vi "test33.vi"() -> ()   [LabVIEW 2021]
uses:
  fft -- waveform manipulate -- control.vi.ctl
  aggregator - viii - real - atomic.vi
  linear interp iiii- real - z-omega.vi
  linear interpolation - real -- V2.vi
  <vilib>/Analysis/baseanly.llb/A x B.vi
  <vilib>/Analysis/baseanly.llb/Real A x B.vi
  Q -- check range -- i -- real.vi
  line -- complex.vi
  Q -- check range -- i -- integer.vi
  Q - not nan -- real.vi
  Q - not nan -- integer.vi
  <vilib>/gmath/interp.llb/Interpolate 1D.vi
  <vilib>/gmath/interp.llb/Search Ordered Table.vi
  <vilib>/Analysis/Matrix/Numeric/Conversions/Array To Matrix.vi
  <vilib>/Analysis/Matrix/Numeric/Conversions/Array To Matrix - RA2.vi
  <vilib>/Analysis/baseanly.llb/Inverse Matrix.vi
  <vilib>/Analysis/baseanly.llb/Real Inverse Matrix.vi
panel:
  in  "times":dbl[](array[numeric]) format="%#_3p"
  out "size(s) 5":i32
  out "size(s) 6":i32
  out "freq vs time 5":cluster{dbl[], dbl[]}(graph)
  out "Array 6":dbl[](array[numeric]) format="%#_3p"
  out "Array 5":dbl[](array[numeric]) format="%#_3p"
  out "freq vs time 4":cluster{dbl[], dbl[]}(graph)
  out "size(s) 3":i32
  out "size(s) 4":i32
  out "Array 4":dbl[](array[numeric]) format="%#_3p"
  out "Array 3":dbl[](array[numeric]) format="%#_3p"
  out "size(s)":i32
  out "size(s) 2":i32
  out "freq vs time 3":cluster{dbl[], dbl[]}[](graph)
  out "Array 2":dbl[](array[numeric]) format="%#_3p"
  out "Array":dbl[](array[numeric]) format="%#_3p"
  out "freq vs time 2":cluster{dbl[], dbl[]}(graph)
  in  "field vs time":cluster{dbl[], dbl[]}(graph)={array[333333 elements], array[333333 elements]}
  in  "freq vs time":cluster{dbl[], dbl[]}(graph)={array[2402 elements], array[2402 elements]}
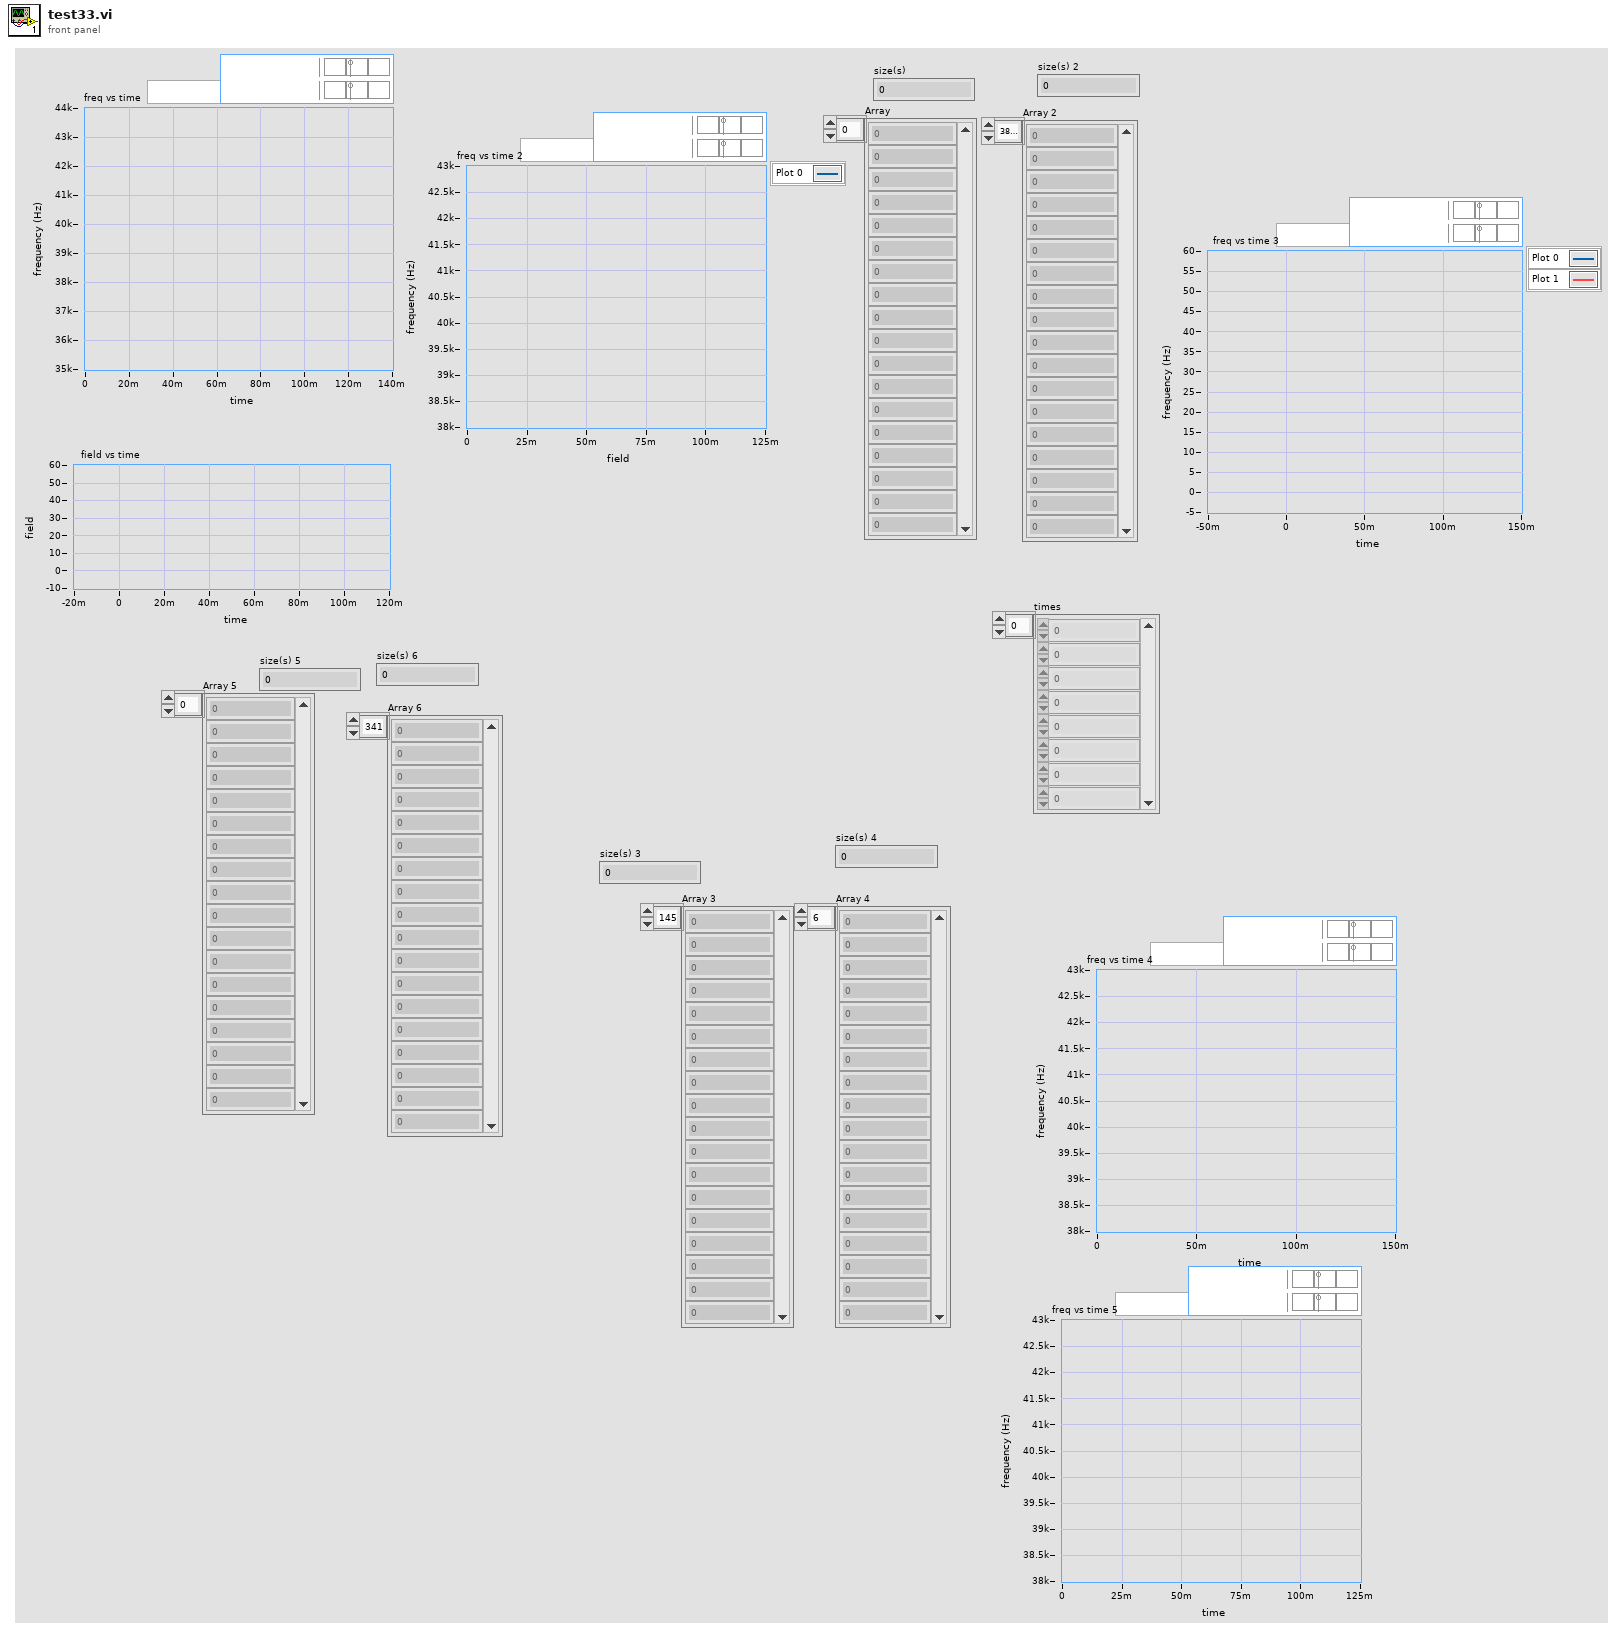
[diagram p1: front panel]
types:
  T1 = typedef "fft -- waveform manipulate -- control.vi.ctl" = enum16{"to array", "to map", "ref from map", "interp from map", "interp from array", "interp other", "delay", "get gamma", "clean 1", "clean 2"}
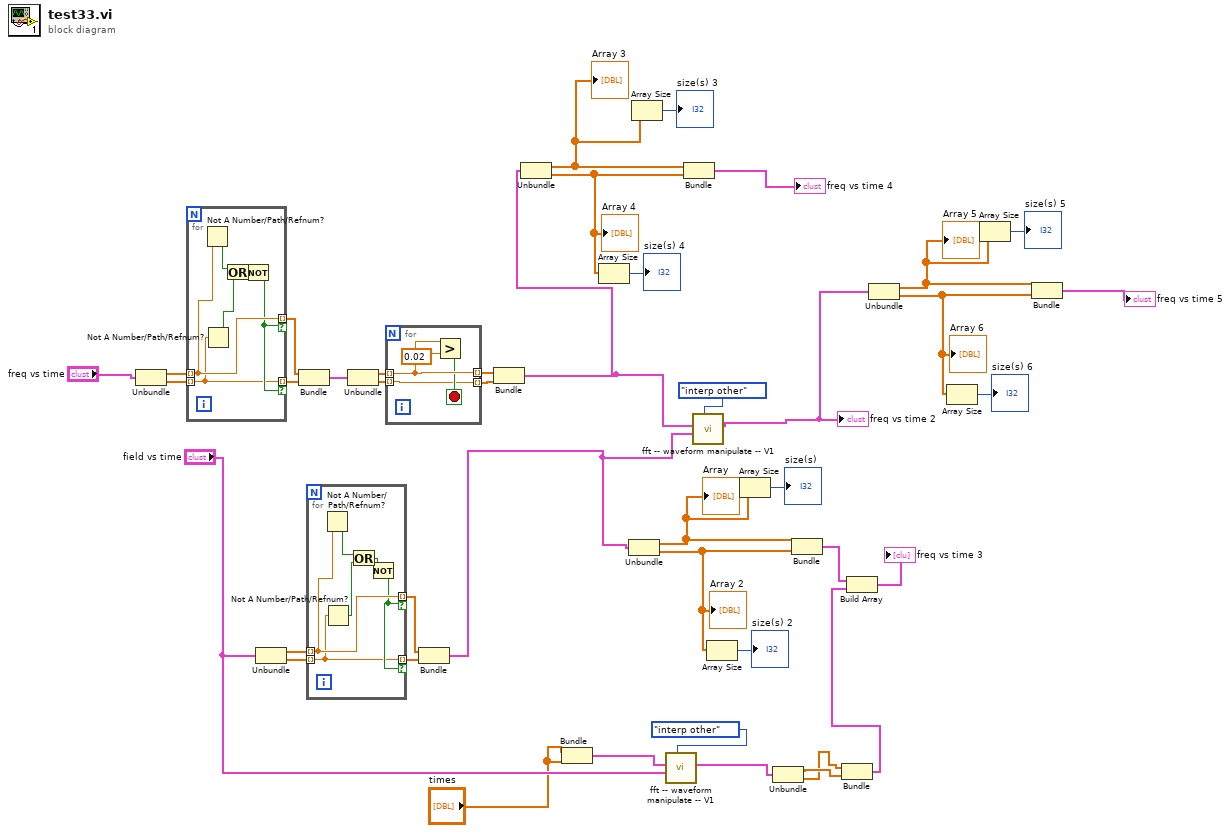
[diagram p0: block diagram]
diagram:
  n1 = Unbundle("freq vs time") -> (w31:dbl[], w30:dbl[])
  n2 = for {
    tunnel: w31 -> [w48] mode=indexing
    tunnel: w30 -> [w43] mode=indexing
    tunnel: [w48] -> w29 mode=indexing if=w44
    tunnel: [w43] -> w28 mode=indexing if=w44
    n3 = Not A Number/Path/Refnum?(number/path/refnum=w48) -> (NaN/Path/Refnum?=w47:bool)
    n4 = Not A Number/Path/Refnum?(number/path/refnum=w43) -> (NaN/Path/Refnum?=w46:bool)
    n5 = Or(x=w47, y=w46) -> (x .or. y?=w45:bool)
    n6 = Not(x=w45) -> (.not. x?=w44:bool)
  }
  n7 = Unbundle("field vs time") -> (w27:dbl[], w26:dbl[])
  n8 = Bundle(w29, w28) -> (w16:cluster{dbl[], dbl[]})  [unwired: 1 in]
  n9 = for {
    tunnel: w27 -> [w54] mode=indexing
    tunnel: w26 -> [w49] mode=indexing
    tunnel: [w54] -> w25 mode=indexing if=w50
    tunnel: [w49] -> w24 mode=indexing if=w50
    n10 = Not A Number/Path/Refnum?(number/path/refnum=w54) -> (NaN/Path/Refnum?=w53:bool)
    n11 = Not A Number/Path/Refnum?(number/path/refnum=w49) -> (NaN/Path/Refnum?=w52:bool)
    n12 = Or(x=w53, y=w52) -> (x .or. y?=w51:bool)
    n13 = Not(x=w51) -> (.not. x?=w50:bool)
  }
  n14 = Unbundle(w16) -> (w15:dbl[], w12:dbl[])
  n15 = for {
    tunnel: [w58] -> w14 mode=indexing
    tunnel: w15 -> [w58] mode=indexing
    tunnel: [w55] -> w13 mode=indexing
    tunnel: w12 -> [w55] mode=indexing
    stop <- w56 stop-if-true
    n16 = Greater?(x=w58, y=0.02) -> (0:w56:bool)
  }
  n17 = Bundle(w25, w24) -> (w23:cluster{dbl[], dbl[]})  [unwired: 1 in]
  n18 = Bundle(w14, w13) -> (w11:cluster{dbl[], dbl[]})  [unwired: 1 in]
  n19 = Unbundle(w11) -> (w34:dbl[], w37:dbl[])
  "Array 3" <- w34
  "Array 4" <- w37
  n20 = Bundle("times"="times", "times"="times") -> (w9:cluster{"times":dbl[], "times":dbl[]})  [unwired: 1 in]
  n21 = Array Size(array=w37) -> (size(s)=→"size(s) 4":i32)
  n22 = Unbundle(w23) -> (w38:dbl[], w41:dbl[])
  "Array" <- w38
  "Array 2" <- w41
  n23 = Array Size(array=w34) -> (size(s)=→"size(s) 3":i32)
  n24 = call "fft -- waveform manipulate -- V1.vi"("fft -- manipulate"=fft_--_waveform_manipulate_--_control.vi."interp other", "Ref Cluster IN"="field vs time", "Cluster IN"=w9) -> ("Cluster out"=w5:cluster{dbl[], dbl[]})  [unwired: 5 in, 3 out]
  n25 = Bundle(w34, w37) -> (→"freq vs time 4":cluster{dbl[], dbl[]})  [unwired: 1 in]
  n26 = call "fft -- waveform manipulate -- V1.vi"("fft -- manipulate"=fft_--_waveform_manipulate_--_control.vi."interp other", "Ref Cluster IN"=w23, "Cluster IN"=w11) -> ("Cluster out"=w17:cluster{dbl[], dbl[]})  [unwired: 5 in, 3 out]
  "freq vs time 2" <- w17
  n27 = Array Size(array=w41) -> (size(s)=→"size(s) 2":i32)
  n28 = Array Size(array=w38) -> (size(s)=→"size(s)":i32)
  n29 = Unbundle(w5) -> (w4:dbl[], w3:dbl[])
  n30 = Bundle(w38, w41) -> (w8:cluster{dbl[], dbl[]})  [unwired: 1 in]
  n31 = Bundle(w3, w4) -> (w2:cluster{dbl[], dbl[]})  [unwired: 1 in]
  n32 = Build Array(w8, w2) -> (→"freq vs time 3":cluster{dbl[], dbl[]}[])
  n33 = Unbundle(w17) -> (w18:dbl[], w21:dbl[])
  "Array 5" <- w18
  "Array 6" <- w21
  n34 = Array Size(array=w21) -> (size(s)=→"size(s) 6":i32)
  n35 = Array Size(array=w18) -> (size(s)=→"size(s) 5":i32)
  n36 = Bundle(w18, w21) -> (→"freq vs time 5":cluster{dbl[], dbl[]})  [unwired: 1 in]
